vi "HFRR ADV v038.vi"() -> ()   [LabVIEW 2025] (continued)
    n1685 = case shown="True" w2039 {
      selector: w2039 -> [_ w2047]
      tunnel: w2037 -> [_ w2048]
      frame False {
      }
      frame True {
        n1686 = Not(x=w2047) -> (.not. x?=w2046:bool)
        n1687 = local write "Calibration Tare"(w2046) -> ()
        "Calibration Tare Value" <- w2048
      }
    }
    n1688 = local read "Quit"() -> (w2045:bool)
  }
  n1689 = while {
    stop <- w2071 stop-if-true
    n1690 = local read "Due read"() -> (w2069:string)
    n1691 = call <vilib>:"High Resolution Polling Wait.vi"("seconds to wait"=0.02) -> ()  [unwired: 10 in, 1 out]
    n1692 = local read "Frictioin Force Raw"() -> (w2051:dbl)
    n1693 = Spreadsheet String To Array(delimiter (Tab)=";", format string="", spreadsheet string=w2069, array type (2D Dbl)=string[] []) -> (array=w2066:string[])
    n1694 = Fract/Exp String To Number(string=w2066) -> (number=w2065:dbl[])  [unwired: 3 in, 1 out]
    n1695 = call <vilib>:"Median Filter PtByPt.vi"("rank"=2, "x"=w2051) -> ("Filtered x"=→"Friction":dbl)  [unwired: 2 in, 1 out]
    n1696 = Index Array(array=w2065) -> (element #1=→"Sample Temperature":dbl, element #2=→"Target Sample Temperature":dbl, element #3=→"Current Duty Cycle":dbl, element #4=→"Ambient Temperature":dbl, element #5=→"Dac Status":dbl, element #6=→"Vpp":dbl, element #7=→"Active Error Code":dbl, element #8=→"Kp":dbl, element #9=→"Ki":dbl, element #10=→"Kd":dbl, element #11=→"SampleRaw":dbl, element #12=→"AmbRaw":dbl)  [unwired: 12 in]
    n1697 = local read "Quit"() -> (w2071:bool)
  }
  n1698 = while {
    shift-right: [w2085] -> w41
    shift-left: _ -> [w2077]
    shift-right: [w2072] -> w40
    shift-left: errorcluster {"status"=FALSE, "code"=0, "source"="Init"} ("error out") -> [w2079]
    tunnel: [w2074] -> w44
    tunnel: [w2084] -> _
    i -> [w2084]
    stop <- w2074 stop-if-true
    n1699 = local read "Com Port 2"() -> (w2078:refnum<visa-resource-name>)
    n1700 = local read "Port 2a"() -> (w2080:bool)
    n1701 = Unbundle(w2079) -> ("status"=→"Port 4":bool)  [unwired: 2 out]
    n1702 = call <vilib>:"High Resolution Polling Wait.vi"("seconds to wait"=0.02) -> ()  [unwired: 10 in, 1 out]
    n1703 = local read "Port 4"() -> (w2081:bool)
    n1704 = Not Equal?(x=w2078, y=w2077) -> (x != y?=w2076:bool)
    n1705 = Or(x=w2081, y=w2080) -> (x .or. y?=w2083:bool)
    n1706 = case shown="False" w2083 {
      frame False {
        w2088 = TRUE ("Visible")
        n1707 = property on="Port 2a" class="Bool (strict)"("Visible"=w2088) -> ()  [unwired: 2 in, 2 out]
        n1708 = property on="Port 4" class="Bool (strict)"("Visible"=w2088) -> ()  [unwired: 2 in, 2 out]
      }
      frame True {
        w2089 = TRUE ("Visible")
        n1709 = property on="Port 2a" class="Bool (strict)"("Visible"=w2089) -> ()  [unwired: 2 in, 2 out]
        n1710 = property on="Port 4" class="Bool (strict)"("Visible"=w2089) -> ()  [unwired: 2 in, 2 out]
      }
    }
    n1711 = case shown="True" w2076 {
      tunnel: [w2086 errorcluster {"status"=TRUE, "code"=0, "source"="Init"} ("error out")] -> w2075
      tunnel: w2079 -> [w2086 _]
      frame False {
      }
      frame True {
      }
    }
    n1712 = case shown="No Error" w2075 {
      selector: w2075 -> [w2102 w2133]
      tunnel: [w2095 w2138] -> w2085
      tunnel: [w2103 w2131] -> w2072
      tunnel: w2077 -> [w2104 w2136]
      frame No Error {
        n1713 = property class="Instr" props=["Serial Settings:Number of Bytes at Serial Port"](reference=w2104, error in=w2102) -> (reference out=w2096:refnum<visa-resource-name>, error out=w2101:errorcluster)  [unwired: 1 out]
        n1714 = while {
          tunnel: [w2112] -> w2097
          tunnel: [w2111] -> w2098
          tunnel: w2101 -> [w2110]
          tunnel: w2096 -> [w2109]
          tunnel: [w2108] -> _
          i -> [w2108]
          stop <- TRUE stop-if-true
          n1715 = property class="Instr" props=["Serial Settings:Number of Bytes at Serial Port"](reference=w2109, error in=w2110) -> (reference out=w2114:refnum<visa-resource-name>, error out=w2113:errorcluster)  [unwired: 1 out]
          n1716 = VISA Read(VISA resource name=w2114, byte count=u32 1000, error in (no error)=w2113) -> (VISA resource name out=w2111:refnum<visa-resource-name>, read buffer=→"Due read":string, error out=w2112:errorcluster)  [unwired: 1 out]
        }
        n1717 = local read "Due Write"() -> (w2094:string)
        n1718 = call <vilib>:"Trim Whitespace.vi"("string"=w2094) -> ("trimmed string"=w2093:string)  [unwired: 1 in]
        n1719 = Not Equal?(x=w2093, y="") -> (x != y?=w2099:bool)
        n1720 = VISA Flush I/O Buffer(VISA resource name=w2098) -> (VISA resource name out=w2091:refnum<visa-resource-name>, error out=→"error out 10":errorcluster)  [unwired: 2 in]
        n1721 = case shown="True" w2099 {
          tunnel: w2091 -> [w2116 w2121]
          tunnel: [w2116 w2125] -> w2095
          tunnel: w2097 -> [w2115 w2120]
          tunnel: [w2115 w2123] -> w2103
          tunnel: w2093 -> [_ w2119]
          tunnel: [_ w2122] -> _
          frame False {
            # "DATA  WRITE LOOP"
          }
          frame True {
            n1722 = Concatenate Strings(w2119, "\r\n") -> (w2118:string)
            n1723 = VISA Write(VISA resource name=w2121, write buffer=w2118, error in (no error)=w2120) -> (VISA resource name out=w2125:refnum<visa-resource-name>, return count=w2122:u32, error out=w2124:errorcluster)
            n1724 = flat-sequence {
              tunnel: w2124 -> [w2127]
              tunnel: [w2127] -> w2123
              frame #0 {
                n1725 = local write "Due Write"("" ("Command")) -> ()
                n1726 = Wait (ms)(milliseconds to wait=u32 5) -> ()  [unwired: 1 out]
              }
            }
          }
        }
        "Port 2a" <- TRUE ("Port 2a")
      }
      frame Error {
        w2144 = u16 0 items=["None", "XON/XOFF", "RTS/CTS", "XON/XOFF & RTS/CTS", "DTR/DSR", "XON/XOFF & DTR/DSR"] ("flow control (0:none)  2")
        w2142 = u16 10 items=["1.0"=10, "1.5"=15, "2.0"=20] ("stop bits 2")
        w2140 = u16 0 items=["None", "Odd", "Even", "Mark", "Space"] ("parity 2")
        w2141 = u32 10000  # timeout (10sec)
        n1727 = VISA Clear(VISA resource name=w2136, error in (no error)=w2133) -> (VISA resource name out=w2135:refnum<visa-resource-name>, error out=w2134:errorcluster)
        n1728 = VISA Close(VISA resource name=w2135, error in (no error)=w2134) -> (error out=w2137:errorcluster)
        n1729 = call <vilib>:"Clear Errors.vi"("error in (no error)"=w2137) -> ()  [unwired: 5 in, 2 out]
        n1730 = local write "Port 2a"(FALSE ("Port 2a")) -> ()
        n1731 = local read "Com Port 2"() -> (w2130:refnum<visa-resource-name>)
        "visa due" <- w2130
        n1732 = call-poly "VISA Configure Serial Port"("VISA resource name"=w2130, "timeout (10sec)"=w2141, "baud rate (9600)"=u32 250000 ("baud rate  2"), "data bits (8)"=u16 8 ("data bits  2"), "parity (0:none)"=w2140, "stop bits (10: 1 bit)"=w2142, "flow control (0:none)"=w2144) -> ("VISA resource name out"=w2145:refnum<visa-resource-name>, "error out"=w2146:errorcluster)  [unwired: 7 in]
        n1733 = flat-sequence {
          tunnel: w2145 -> [w2148]
          tunnel: w2146 -> [w2147]
          tunnel: [w2148] -> w2138
          tunnel: [w2147] -> w2131
          frame #0 {
            n1734 = Wait (ms)(milliseconds to wait=u32 50) -> ()  [unwired: 1 out]
          }
        }
        "Residual Due" <- ""
      }
    }
    "error out 9" <- w2072
    n1735 = local read "Quit"() -> (w2074:bool)
    "Error Due" <- w2079
  }
  n1736 = local write "FRICVALZ"(0.0 ("FRICVALZ")) -> ()
  n1737 = property on="RUN" class="Bool (strict)"("Visible"=TRUE) -> ()  [unwired: 2 in, 2 out]
  n1738 = while {
    tunnel: [w2163] -> _
    tunnel: [w2150] -> w54
    i -> [w2163]
    stop <- w2150 stop-if-true
    n1739 = local read "conststatus"() -> (w2154:dbl)
    n1740 = local read "Main Tab"() -> (w2152:T2)
    n1741 = local read "EDIT"() -> (w2169:bool)
    n1742 = local read "Rate"() -> (w2168:dbl)
    n1743 = case shown="True" w2169 {
      tunnel: [FALSE TRUE] -> _
      frame False {
      }
      frame True {
      }
    }
    n1744 = Equal?(x=w2152, y=T29."About" ("Main Tab")) -> (x = y?=w2161:bool)
    n1745 = Equal?(x=w2154, y=0.0) -> (x = y?=w2155:bool)
    n1746 = Divide(x=1.0, y=w2168) -> (x/y=w2164:dbl)
    "Time 2" <- w2164
    n1747 = case shown="True" w2155 {
      frame False {
      }
      frame True {
        # "C:\\WinDucom\\calibrate WO 2391.dcf"
        n1748 = local write "Lan flag"(22) -> ()
        n1749 = local write "conststatus"(10.0 ("rpm value : 2")) -> ()
        n1750 = String To Path(string="C:\\LAB-IQ\\calibrate WO 2465.dcf") -> (path=w2175:path)
        n1751 = Open/Create/Replace File "Open File"(file path (use dialog)=w2175) -> (refnum out=w2173:refnum<file>)  [unwired: 5 in, 2 out]
        n1752 = for {
          N: 23 -> [_]
          tunnel: w2173 -> [w2184]
          i -> [w2178]
          (unwired) TRUE ("line mode (F)")
          n1753 = Read from Text File "Read File"(file (use dialog)=w2184) -> (text=w2183:string)  [unwired: 3 in, 3 out]
          n1754 = Match Pattern(string=w2183, regular expression="]") -> (after substring=w2181:string)  [unwired: 1 in, 3 out]
          n1755 = String Subset(string=w2183, offset (0)=5, length (rest)=10 ("length (rest)")) -> (substring=w2176:string)
          n1756 = Fract/Exp String To Number(string=w2176) -> (number=w2177:dbl)  [unwired: 3 in, 1 out]
          n1757 = Match Pattern(string=w2181, regular expression="-") -> (before substring=w2179:string)  [unwired: 1 in, 3 out]
          n1758 = case shown="10" w2178 {
            tunnel: w2177 -> [_ _ _ _ _ _ _ _ _ _ w2191 _ _ _ _ _ _ _ _ _ _ _ _ _]
            tunnel: w2179 -> [_ _ _ _ w2187 w2188 w2189 _ _ _ _ _ _ _ _ _ _ _ _ _ w2192 w2193 w2194 _]
            frame 0 {
            }
            frame 1 {
            }
            frame 2 {
            }
            frame 3 {
            }
            frame 4 {
              n1759 = local write "Com Port 1"(w2187) -> ()
            }
            frame 5 {
              n1760 = local write "Com Port 2"(w2188) -> ()
              n1761 = local write "visa due"(w2188) -> ()
            }
            frame 6 {
              n1762 = String To Path(string=w2189) -> (path=w2190:path)
              n1763 = local write "File Path"(w2190) -> ()
              "String" <- w2189
            }
            frame 7 {
            }
            frame 8 {
            }
            frame 9 {
            }
            frame 10 {
              n1764 = local write "Language Selection"(w2191) -> ()
            }
            frame 11 {
            }
            frame 12 {
            }
            frame 13 {
            }
            frame 14 {
            }
            frame 15 {
            }
            frame 16 {
            }
            frame 17 {
            }
            frame 18 {
            }
            frame 21 {
            }
            frame 22 {
              n1765 = local write "Com Port 3"(w2192) -> ()
            }
            frame 20 {
              n1766 = local write "Camera Port :"(w2193) -> ()
            }
            frame 19 {
              n1767 = local write "C3 :"(w2194) -> ()
            }
            frame 23, Default {
            }
          }
        }
      }
    }
    n1768 = Select(t=u32 2500 ("milliseconds to wait"), s=w2161, f=u32 500 ("milliseconds to wait")) -> (s? t:f=w2159:u32)
    n1769 = Multiply(x=w2164, y=w2159) -> (x*y=w2166:dbl)
    n1770 = call "Elapsed Time2"("Time Target (s)"=w2166, "Auto Reset"=TRUE) -> ("Time has Elapsed"=w2156:bool)  [unwired: 10 in, 7 out]
    n1771 = case shown="True" w2156 {
      frame False {
      }
      frame True {
        n1772 = stacked-sequence {
          frame #0 {
            # "DATA PROCESSING"
            # "115 mV/N"
            n1773 = local read "Sample Temperature"() -> (w2197:dbl)
            n1774 = local read "RH Numeric:"() -> (→"Humidity ( %RH )":dbl)
            n1775 = local read "FRICVALZ"() -> (w2214:dbl)
            n1776 = local read "Friction"() -> (w2200:dbl)
            n1777 = call <vilib>:"Mean PtByPt.vi"("x"=w2197, "sample length"=100) -> ("mean"=w2196:dbl)  [unwired: 2 in, 1 out]
            "TEMP 2" <- w2196
            "TEMP 3" <- w2196
            n1778 = Subtract(x=w2200, y=w2214) -> (x-y=w2209:dbl)
            "FF 2" <- w2209
            "FF 4" <- w2209
            n1779 = local read "Ambient Temperature"() -> (→"AIR TEMP":dbl)
            n1780 = local read "TEMP"() -> (w2213:dbl)
            n1781 = local write "FF 3"(w2209) -> ()
            n1782 = Compound Arithmetic op=OR("FRICVALZ 4", "FRICVALZ 3", "FRICVALZ 2") -> (w2205:bool)
            n1783 = case shown="True" w2205 {
              tunnel: w2200 -> [_ w2220]
              frame False {
              }
              frame True {
                w2219 = FALSE ("FRICVALZ")
                n1784 = local write "FRICVALZ 3"(w2219) -> ()
                n1785 = local write "FRICVALZ 2"(w2219) -> ()
                n1786 = local write "FRICVALZ 4"(w2219) -> ()
                "FRICVALZ" <- w2220
              }
            }
            n1787 = Not A Number/Path/Refnum?(number/path/refnum=w2213) -> (NaN/Path/Refnum?=w2212:bool)
            n1788 = Not A Number/Path/Refnum?(number/path/refnum=w2209) -> (NaN/Path/Refnum?=w2211:bool)
            n1789 = Divide(x=w2209, y=1.96) -> (x/y=w2206:dbl)
            n1790 = Compound Arithmetic op=OR(w2212, w2211) -> (w2210:bool)
            n1791 = Not A Number/Path/Refnum?(number/path/refnum=w2206) -> (NaN/Path/Refnum?=w2207:bool)
            n1792 = case shown="True" w2210 {
              frame False {
              }
              frame True {
                n1793 = local write "TEMP"(0.0 ("TEMP")) -> ()
                n1794 = local write "FF 2"(0.0 ("FF 2")) -> ()
                n1795 = local write "reinit"(TRUE ("reinit")) -> ()
              }
            }
            n1796 = local write "TEMP"(w2196) -> ()
            n1797 = Select(t=0.0, s=w2207, f=w2206) -> (s? t:f=w2199:dbl)
            "COF 2" <- w2199
            n1798 = local write "COF 3"(w2199) -> ()
          }
        }
      }
    }
    n1799 = Wait (ms)(milliseconds to wait=u32 50) -> ()  [unwired: 1 out]
    n1800 = local read "Quit"() -> (w2150:bool)
    "Rate" <- 2500.0 ("No of Samples")
  }
  n1801 = while {
    tunnel: [w2240] -> _
    tunnel: [w2223] -> w56
    tunnel: w1 -> [_]
    i -> [w2240]
    stop <- w2223 stop-if-true
    # "C:\\LAB-IQ-NXT\\Scar View.exe"
    n1802 = local read "OK Button 16"() -> (w2230:bool)
    n1803 = local read "Main Tab"() -> (w2224:T2)
    n1804 = local read "service 3"() -> (w2225:bool)
    n1805 = local read "OPEN 6"() -> (w2227:bool)
    n1806 = local read "EDIT 2"() -> (w2229:bool)
    n1807 = flat-sequence {
      frame #0 {
        n1808 = stacked-sequence {
          frame #0 {
            n1809 = local read "EDIT"() -> (w2718:bool)
            n1810 = case shown="False" w2718 {
              tunnel: [u8 2 ("Disabled") u8 0 ("Disabled")] -> _
              frame False {
                w2720 = FALSE
                n1811 = local write "Password"("") -> ()
                n1812 = local write "x = y?"(w2720) -> ()
                n1813 = property on="Password" class="Str"("Visible"=w2720) -> ()  [unwired: 2 in, 2 out]
              }
              frame True {
                n1814 = property on="Password" class="Str"("Visible"=TRUE) -> ()  [unwired: 2 in, 2 out]
              }
            }
            "dipl pwd" <- "@143$\n" ("dipl pwd")
          }
          frame #1 {
          }
          frame #2 {
          }
          frame #3 {
          }
          frame #4 {
            n1815 = String To Byte Array(string="Password") -> (unsigned byte array=w2731:u8[])
            n1816 = Search 1D Array(1D array=w2731, element=u8 10) -> (index of element=w2729:i32)  [unwired: 1 in]
            n1817 = Index Array(array=w2731, index=w2729) -> (element=w2730:u8)
            n1818 = Equal?(x=w2730, y=10) -> (x = y?=w2726:bool)
            n1819 = case shown="True" w2726 {
              frame False {
              }
              frame True {
                # "password"
                # "password"
                n1820 = local read "Password"() -> (w2743:string)
                n1821 = String To Byte Array(string=w2743) -> (unsigned byte array=w2746:u8[])
                n1822 = String To Byte Array(string="@143$\n") -> (unsigned byte array=w2733:u8[])
                n1823 = Array Size(array=w2746) -> (size(s)=w2742:i32)
                n1824 = Array Size(array=w2733) -> (size(s)=w2738:i32)
                n1825 = for {
                  N: w2742 -> [_]
                  tunnel: w2746 -> [w2759]
                  tunnel: [w2757] -> w2747 mode=indexing
                  tunnel: w2742 -> [w2754]
                  i -> [w2755]
                  n1826 = Decrement(x=w2754) -> (x-1=w2753:i32)
                  n1827 = Index Array(array=w2759, index=w2755) -> (element=w2758:u8)
                  n1828 = Equal?(x=w2755, y=w2753) -> (x = y?=w2752:bool)
                  n1829 = Number To Decimal String(number=w2758) -> (decimal integer string=w2756:string)  [unwired: 1 in]
                  n1830 = Select(t="", s=w2752, f="\r") -> (s? t:f=w2749:string)
                  n1831 = Concatenate Strings(w2756, w2749) -> (w2757:string)
                }
                n1832 = for {
                  N: w2738 -> [_]
                  tunnel: w2733 -> [w2770]
                  tunnel: [w2768] -> w2736 mode=indexing
                  tunnel: w2738 -> [w2765]
                  i -> [w2766]
                  n1833 = Decrement(x=w2765) -> (x-1=w2764:i32)
                  n1834 = Index Array(array=w2770, index=w2766) -> (element=w2769:u8)
                  n1835 = Equal?(x=w2766, y=w2764) -> (x = y?=w2763:bool)
                  n1836 = Number To Decimal String(number=w2769) -> (decimal integer string=w2767:string)  [unwired: 1 in]
                  n1837 = Select(t="", s=w2763, f="\r") -> (s? t:f=w2760:string)
                  n1838 = Concatenate Strings(w2767, w2760) -> (w2768:string)
                }
                n1839 = local read "file path"() -> (w2732:path)
                n1840 = call <vilib>:"Read Characters From File.vi"("file path (dialog if empty)"=w2732) -> ("character string"=w2745:string)  [unwired: 5 in, 3 out]
                "string" <- w2745
                n1841 = flat-sequence {
                  tunnel: [w2748] -> _
                  frame #0 {
                    w2748 = ""
                    n1842 = local write "Password"(w2748) -> ()
                  }
                }
                n1843 = Concatenate Strings(w2736) -> (w2737:string)
                n1844 = Concatenate Strings(w2745) -> (w2744:string)
                n1845 = Concatenate Strings(w2747) -> (w2740:string)
                n1846 = Equal?(x=w2740, y=w2744) -> (x = y?=w2735:bool)
                n1847 = Equal?(x=w2740, y=w2737) -> (x = y?=w2741:bool)
                n1848 = Or(x=w2735, y=w2741) -> (x .or. y?=→"x = y?":bool)
              }
            }
          }
        }
        n1849 = local read "x = y?"() -> (w2716:bool)
        n1850 = And(x="EDIT", y=w2716) -> (x .and. y?=w2714:bool)
        n1851 = case shown="True" w2714 {
          tunnel: [u8 2 ("Disabled") u8 0 ("Disabled")] -> w2713
          tunnel: [w2920 TRUE ("Visible")] -> w2712
          frame False {
            w2920 = FALSE ("Visible")
            n1852 = local write "EDIT 2"(w2920) -> ()
          }
          frame True {
          }
        }
        n1853 = case shown="True" "SAVE" {
          frame False {
          }
          frame True {
            n1854 = stacked-sequence {
              seq-local: [w2775 _ _] -> [_ w2916 _]
              frame #0 {
                w2771 = 0.0 ("number")
                w2772 = 0.0 ("number")
                (unwired) i16 5 ("precision (6)")
                # "[CH1]    - FF\n[CH2]   - TEMPERATURE\n[CH3]    - Humidity\n[CH4]    - AIR TEMP\n[CH5]\\- Visa Uno\n[CH6] \\- Visa Due\n[CH7]  \\- file path\n[CH8]   - Displacement Gain\n[CHA]   - Stroke Gain\n[CHB]   - Stroke PID Gain\n[CHC]   -Language Selection\n[CHD]   -Power +\n[CHE]   -Power_\n[CHF]   -Heater\n[CHG]   -Humidity Wet\n[CHH]   -Humidity Dry\n[CHI]   -Integral Time"
                n1855 = local read "Language Selection"() -> (w2818:enum16{"English", "Russian"})
                n1856 = Path To String(path="File Path") -> (string=w2834:string)
                n1857 = Number To Fractional String(number=w2771, width (-)=i16 10 ("precision (6)"), precision (6)=i16 5) -> (F-format string=w2825:string)  [unwired: 1 in]
                n1858 = Number To Fractional String(number=w2818, width (-)=i16 10 ("precision (6)"), precision (6)=i16 5) -> (F-format string=w2814:string)  [unwired: 1 in]
                n1859 = Number To Fractional String(number=w2772, width (-)=i16 10 ("precision (6)"), precision (6)=i16 5) -> (F-format string=w2808:string)  [unwired: 1 in]
                n1860 = Number To Fractional String(number=w2772, width (-)=i16 10 ("precision (6)"), precision (6)=i16 5) -> (F-format string=w2805:string)  [unwired: 1 in]
                n1861 = Number To Fractional String(number=w2772, width (-)=i16 10 ("precision (6)"), precision (6)=i16 5) -> (F-format string=w2800:string)  [unwired: 1 in]
                n1862 = Number To Fractional String(number=w2772, width (-)=i16 10 ("precision (6)"), precision (6)=i16 5) -> (F-format string=w2797:string)  [unwired: 1 in]
                n1863 = Number To Fractional String(number=w2772, width (-)=i16 10 ("precision (6)"), precision (6)=i16 5) -> (F-format string=w2792:string)  [unwired: 1 in]
                n1864 = local read "Com Port 1"() -> (w2774:refnum<visa-resource-name>)
                n1865 = local read "Com Port 2"() -> (w2773:refnum<visa-resource-name>)
                n1866 = Concatenate Strings(w2834, "\\" ("string")) -> (w2833:string)
                n1867 = Number To Fractional String(number=w2771, width (-)=i16 10 ("precision (6)"), precision (6)=i16 5) -> (F-format string=w2866:string)  [unwired: 1 in]
                n1868 = Number To Fractional String(number=w2771, width (-)=i16 10 ("precision (6)"), precision (6)=i16 5) -> (F-format string=w2865:string)  [unwired: 1 in]
                n1869 = Number To Fractional String(number=w2771, width (-)=i16 10 ("precision (6)"), precision (6)=i16 5) -> (F-format string=w2859:string)  [unwired: 1 in]
                n1870 = Number To Fractional String(number=w2771, width (-)=i16 10 ("precision (6)"), precision (6)=i16 5) -> (F-format string=w2853:string)  [unwired: 1 in]
                n1871 = Number To Fractional String(number=w2771, width (-)=i16 10 ("precision (6)"), precision (6)=i16 5) -> (F-format string=w2826:string)  [unwired: 1 in]
                n1872 = Concatenate Strings("[CHA]" ("string"), w2825, "- Stroke Gain" ("string"), "\r") -> (w2819:string)
                n1873 = Concatenate Strings("[CHC]" ("string"), w2814, "-Language Selection" ("string"), "\r") -> (w2811:string)
                n1874 = Concatenate Strings("[CHD]" ("string"), w2808, "-Power +" ("string"), "\r") -> (w2790:string)
                n1875 = Concatenate Strings("[CHG]" ("string"), w2797, "-Humidity Wet" ("string"), "\r") -> (w2787:string)
                n1876 = Concatenate Strings("[CHH]" ("string"), w2792, "-Humidity Dry" ("string"), "\r") -> (w2786:string)
                n1877 = Concatenate Strings("[CH1]" ("string"), w2866, " - FF" ("string"), "\r") -> (w2864:string)
                n1878 = Concatenate Strings("[CH2]" ("string"), w2865, " - TEMPERATURE" ("string"), "\r") -> (w2863:string)
                n1879 = Concatenate Strings("[CH3]" ("string"), w2859, " - Humidity" ("string"), "\r") -> (w2856:string)
                n1880 = Concatenate Strings("[CH4]" ("string"), w2853, " - AIR TEMP" ("string"), "\r") -> (w2849:string)
                n1881 = Concatenate Strings("[CH5]" ("string"), w2774, "- Visa Uno" ("string"), "\r") -> (w2842:string)
                n1882 = Concatenate Strings("[CH6]" ("string"), w2773, "- Visa Due" ("string"), "\r") -> (w2837:string)
                n1883 = Concatenate Strings("[CH7]" ("string"), w2833, "- file path" ("string"), "\r") -> (w2836:string)
                n1884 = Concatenate Strings("[CH8]" ("string"), w2826, "- Displacement Gain" ("string"), "\r") -> (w2829:string)
                n1885 = Concatenate Strings("[CHE]" ("string"), w2805, "-Power_" ("string"), "\r") -> (w2789:string)
                n1886 = Concatenate Strings("[CHF]" ("string"), w2800, "-Heater" ("string"), "\r") -> (w2788:string)
                n1887 = Concatenate Strings(w2864, w2863, w2856, w2849, w2842, w2837, w2836, w2829, w2819, w2811, w2790, w2789, w2788, w2787, w2786) -> (w2775:string)
                "gain" <- w2775
              }
              frame #1 {
                w2877 = 0.0 ("number")
                n1888 = local read "Camera Port :"() -> (w2880:string)
                n1889 = local read "C3 :"() -> (w2888:refnum<visa-resource-name>)
                n1890 = local read "Com Port 3"() -> (w2889:refnum<visa-resource-name>)
                n1891 = Concatenate Strings("[CH8]" ("string"), w2880, "- Visa Camera" ("string"), "\r") -> (w2879:string)
                n1892 = Concatenate Strings("[CH7]" ("string"), w2888, "- Visa Humidity" ("string"), "\r") -> (w2884:string)
                n1893 = Number To Fractional String(number=w2877, width (-)=i16 10 ("precision (6)"), precision (6)=i16 5) -> (F-format string=w2904:string)  [unwired: 1 in]
                n1894 = Concatenate Strings("[CHL]" ("string"), w2889, "- Visa humid" ("string"), "\r") -> (w2892:string)
                n1895 = Number To Fractional String(number=w2877, width (-)=i16 10 ("precision (6)"), precision (6)=i16 5) -> (F-format string=w2911:string)  [unwired: 1 in]
                n1896 = Concatenate Strings("[CHK]" ("string"), w2904, "-TEMP INTERCEPT" ("string"), "\r") -> (w2900:string)
                n1897 = Concatenate Strings("[SNO]" ("string"), "" ("string"), "-" ("string"), "\r") -> (w2897:string)
                n1898 = Concatenate Strings("[CHJ]" ("string"), w2911, "-AIR TEMP INTERCEPT" ("string"), "\r") -> (w2901:string)
                n1899 = String To Path(string="C:\\LAB-IQ\\calibrate WO 2465.dcf") -> (path=w2890:path)
                n1900 = Concatenate Strings(w2916, w2901, w2900, w2897, w2892, w2884, w2879) -> (w2915:string)
                n1901 = call <vilib>:"Write Characters To File.vi"("append to file? (new file:F)"=FALSE, "character string"=w2915, "file path (dialog if empty)"=w2890) -> ()  [unwired: 2 in, 1 out]
              }
              frame #2 {
                n1902 = local write "Lan flag"(0.0 ("Lan flag")) -> ()
                n1903 = local write "conststatus"(0.0 ("rpm value : 2")) -> ()
                n1904 = local write "SAVE"(FALSE ("OK Button 14")) -> ()
              }
            }
          }
        }
        n1905 = property on="EDIT 2" class="Bool (strict)"("Visible"=w2712) -> ()  [unwired: 2 in, 2 out]
        n1906 = property on="SAVE" class="Bool (strict)"("Visible"=w2712) -> ()  [unwired: 2 in, 2 out]
        n1907 = property on="visa due" class="CmbBox"("Disabled"=w2713) -> ()  [unwired: 2 in, 2 out]
        n1908 = property on="File Path" class="Path"("Disabled"=w2713) -> ()  [unwired: 2 in, 2 out]
        n1909 = property on="Language Selection" class="Enum (strict)"("Visible"=w2712) -> ()  [unwired: 2 in, 2 out]
        n1910 = property on="SPEED OUT:" class="DigNum (strict)"("Disabled"=w2713) -> ()  [unwired: 2 in, 2 out]
      }
    }
    n1911 = local read "RUN"() -> (w2239:bool)
    n1912 = local read "RUN"() -> (w2237:bool)
    n1913 = case shown="True" "EDIT 3" {
      frame False {
      }
      frame True {
        n1914 = local write "EDIT 3"(FALSE ("EDIT 3")) -> ()
        n1915 = local write "Main Tab"(T2."About" ("Main Tab")) -> ()
      }
    }
    n1916 = case shown="False" w2239 {
      frame False {
        n1917 = local read "stopT"() -> (w2927:bool)
        n1918 = case shown="True" w2927 {
          frame False {
          }
          frame True {
            n1919 = local write "stopT"(FALSE) -> ()
          }
        }
      }
      frame True {
        "stopT" <- TRUE
      }
    }
    n1920 = case shown="False" w2237 {
      frame False {
      }
      frame True {
      }
    }
    n1921 = case shown="True" w2229 {
      frame False {
        n1922 = property on="Password 2" class="Str"("Visible"=FALSE) -> ()  [unwired: 2 in, 2 out]
        n1923 = local write "Password 2"("" ("Password")) -> ()
      }
      frame True {
        n1924 = property on="Password 2" class="Str"("Visible"=TRUE) -> ()  [unwired: 2 in, 2 out]
        n1925 = Equal?(x="Password 2", y="HFRR1234") -> (x = y?=w2252:bool)
        n1926 = case shown="True" w2252 {
          tunnel: "Password 2" -> [w2255 _]
          frame False {
            n1927 = String Length(string=w2255) -> (length=w2256:i32)
            n1928 = Greater Than 0?(x=w2256) -> (x > 0?=w2254:bool)
            n1929 = case shown="False" w2254 {
              frame False {
                n1930 = property on="Password 2" class="Str"("Caption.Text"="Password (Advance Setting)") -> ()  [unwired: 2 in, 2 out]
              }
              frame True {
                n1931 = property on="Password 2" class="Str"("Caption.Text"="Incorrect Password!") -> ()  [unwired: 2 in, 2 out]
              }
            }
          }
          frame True {
            n1932 = local write "EDIT 2"(FALSE ("EDIT 2")) -> ()
            n1933 = local write "Password 2"("" ("Password")) -> ()
            n1934 = local write "Main Tab"(T2."Advance" ("Main Tab")) -> ()
            n1935 = local write "Main Dashboard Buttons"(T1."Advance" ("Main Dashboard Buttons")) -> ()
          }
        }
      }
    }
    n1936 = case shown="True" "Prog Uno" {
      frame False {
      }
      frame True {
        n1937 = stacked-sequence {
          frame #0 {
            n1938 = Delete(path (use dialog)=path "C:/LAB-IQ-NXT/UNOCOMPILE.bat" ("working directory")) -> ()  [unwired: 4 in, 3 out]
          }
          frame #1 {
            n1939 = local read "Com Port 1"() -> (w2694:refnum<visa-resource-name>)
            n1940 = Concatenate Strings("cmd.exe /c \"mode " ("command line"), w2694, ":1200,n,8,1\"\n" ("command line")) -> (w2699:string)
            n1941 = Concatenate Strings(w2699, "CD\\\nCD WinDucom\navrdude -C avrdude.conf -v -patmega328p -carduino -P" ("command line"), w2694, " -b115200 -D -Uflash:w:UNO_V20.hex:i\n" ("command line"), "\r") -> (w2701:string)
            "STR" <- w2701
            n1942 = call <vilib>:"Write Characters To File.vi"("append to file? (new file:F)"=FALSE, "character string"=w2701, "file path (dialog if empty)"=path "C:/LAB-IQ/UNOCOMPILE.bat" ("working directory")) -> ()  [unwired: 2 in, 1 out]
          }
          frame #2 {
            n1943 = disable-structure shown="Disabled" {
              frame Disabled {
                w2705 = "cmd.exe  /c \"C:\\LAB-IQ-NXT\\UNOCOMPILE.bat\"" ("string")
                n1944 = local write "Prog Uno"(FALSE ("run minimized? (F)")) -> ()
                n1945 = call <vilib>:"System Exec.vi"("expected output size  (4096)"=u32 65535, "run minimized? (F)"=FALSE, "wait until completion? (T)"=TRUE ("run minimized? (F)"), "working directory"=path "C:/LAB-IQ-NXT", "standard input"=w2705, "command line"=w2705) -> ("error out"=w2704:errorcluster, "standard output"=→"String 42":string)  [unwired: 2 in, 2 out]
                "error out 3" <- w2704
                n1946 = flat-sequence {
                  tunnel: w2704 -> [_]
                  frame #0 {
                  }
                }
              }
              frame Enabled {
              }
            }
          }
        }
      }
    }
    n1947 = case shown="\"ISO 12156\"" "TEST STANDARD" {
      frame "ASTM D6079", Default {
        w2674 = 50.0 ("Hz")
        w2675 = 53.0 ("Set Rh")
        w2677 = 1.0 ("Set Strk")
        w2676 = 60.0 ("Set Temp")
        # "astm hide"
        n1948 = local write "NORMAL LOAD"(200.0 ("NORMAL LOAD")) -> ()
        n1949 = local write "Set Strk"(w2677) -> ()
        n1950 = local write "Set Hz"(w2674) -> ()
        n1951 = local write "Set Temp"(w2676) -> ()
        n1952 = local write "Set Rh"(w2675) -> ()
        n1953 = local write "test time"(75.0 ("test time")) -> ()
        n1954 = local write "Set Stroke:"(w2677) -> ()
        n1955 = local write "Set Humidity:"(w2675) -> ()
        n1956 = local write "Set Frequency:"(w2674) -> ()
        n1957 = local write "Set Temperature:"(w2676) -> ()
        "Test Standard" <- "ASTM D6079" ("Test Standard 2")
      }
      frame "ISO 12156" {
        n1958 = local write "Set Strk"(1.0 ("Set Strk")) -> ()
        n1959 = local write "NORMAL LOAD"(200.0 ("NORMAL LOAD")) -> ()
        n1960 = local write "Set Temp"(60.0 ("Set Temp")) -> ()
        n1961 = local write "test time"(75.0 ("test time")) -> ()
        n1962 = local write "Set Hz"(50.0 ("Hz")) -> ()
        n1963 = local write "Set Rh"(53.0 ("Set Rh")) -> ()
      }
      frame "CEC F-096-A-06" {
        n1964 = local write "Set Strk"(1.0 ("Set Strk")) -> ()
        n1965 = local write "NORMAL LOAD"(200.0 ("NORMAL LOAD")) -> ()
        n1966 = local write "Set Temp"(60.0 ("Set Temp")) -> ()
        n1967 = local write "test time"(75.0 ("test time")) -> ()
        n1968 = local write "Set Hz"(50.0 ("Hz")) -> ()
        n1969 = local write "Set Rh"(53.0 ("Set Rh")) -> ()
      }
      frame "Custom" {
      }
    }
    n1970 = Or(x=w2227, y=w2225) -> (x .or. y?=w2226:bool)
    n1971 = case shown="\"About\"" w2224 {
      tunnel: [T29."Acquire" ("Main Tab") T29."Compare Files" ("Main Tab") T29."About" ("Main Tab")] -> w2235
      frame "Acquire", Default {
      }
      frame "Compare Files" {
      }
      frame "About" {
      }
    }
    n1972 = Or(x=w2230, y="OPEN") -> (x .or. y?=w2231:bool)
    n1973 = case shown="True" w2231 {
      tunnel: w2230 -> [_ w2263]
      frame False {
      }
      frame True {
        n1974 = stacked-sequence {
          tunnel: w2263 -> [_ w2330 _ _]
          frame #0 {
            w2279 = "  " ("String 6")
            n1975 = local write "OPEN"(FALSE ("open")) -> ()
            n1976 = local read "string1 2"() -> (w2267:string)
            n1977 = local read "string1 3"() -> (w2266:string)
            n1978 = local read "string1 4"() -> (w2265:string)
            n1979 = property on="OPEN" class="Bool (strict)"("Visible"=FALSE) -> ()  [unwired: 2 in, 2 out]
            n1980 = local write "String 6"(w2279) -> ()
            n1981 = local write "String 7"(w2279) -> ()
            n1982 = local write "String 8"(w2279) -> ()
            n1983 = local write "String 12"(w2279) -> ()
            n1984 = local read "OK Button 16"() -> (w2264:bool)
            n1985 = String To Path(string=w2267) -> (path=w2275:path)
            n1986 = String To Path(string=w2266) -> (path=w2274:path)
            n1987 = String To Path(string=w2265) -> (path=w2273:path)
            n1988 = case shown="True" w2264 {
              tunnel: [w2280 w2281] -> w2268
              frame False {
                n1989 = local read "string1"() -> (w2280:string)
              }
              frame True {
                n1990 = local read "String Indicator 4"() -> (w2281:string)
              }
            }
            n1991 = Open/Create/Replace File "Open File"(file path (use dialog)=w2275) -> (refnum out=w2271:refnum<file>)  [unwired: 5 in, 2 out]
            n1992 = Open/Create/Replace File "Open File"(file path (use dialog)=w2274) -> (refnum out=w2270:refnum<file>)  [unwired: 5 in, 2 out]
            n1993 = Open/Create/Replace File "Open File"(file path (use dialog)=w2273) -> (refnum out=w2269:refnum<file>)  [unwired: 5 in, 2 out]
            n1994 = while {
              tunnel: w2271 -> [w2293]
              i -> [w2289]
              stop <- w2288 continue-if-true
              (unwired) TRUE ("line mode (F)")
              n1995 = Read from Text File "Read File"(file (use dialog)=w2293) -> (text=w2290:string)  [unwired: 3 in, 3 out]
              n1996 = local write "Numeric 11"(w2289) -> ()
              n1997 = String Length(string=w2290) -> (length=w2292:i32)
              n1998 = Greater?(x=w2292, y=1) -> (0:w2288:bool)
            }
            n1999 = while {
              tunnel: w2270 -> [w2299]
              i -> [w2295]
              stop <- w2294 continue-if-true
              (unwired) TRUE ("line mode (F)")
              n2000 = Read from Text File "Read File"(file (use dialog)=w2299) -> (text=w2296:string)  [unwired: 3 in, 3 out]
              n2001 = local write "Numeric 12"(w2295) -> ()
              n2002 = String Length(string=w2296) -> (length=w2298:i32)
              n2003 = Greater?(x=w2298, y=1) -> (0:w2294:bool)
            }
            n2004 = while {
              tunnel: w2269 -> [w2305]
              i -> [w2301]
              stop <- w2300 continue-if-true
              (unwired) TRUE ("line mode (F)")
              n2005 = Read from Text File "Read File"(file (use dialog)=w2305) -> (text=w2302:string)  [unwired: 3 in, 3 out]
              n2006 = local write "Numeric 13"(w2301) -> ()
              n2007 = String Length(string=w2302) -> (length=w2304:i32)
              n2008 = Greater?(x=w2304, y=1) -> (0:w2300:bool)
            }
            n2009 = String To Path(string=w2268) -> (path=w2276:path)
            n2010 = Open/Create/Replace File "Open File"(file path (use dialog)=w2276) -> (refnum out=w2272:refnum<file>)  [unwired: 5 in, 2 out]
            n2011 = while {
              tunnel: w2272 -> [w2287]
              i -> [w2283]
              stop <- w2282 continue-if-true
              (unwired) TRUE ("line mode (F)")
              n2012 = Read from Text File "Read File"(file (use dialog)=w2287) -> (text=w2284:string)  [unwired: 3 in, 3 out]
              n2013 = local write "Numeric 8"(w2283) -> ()
              n2014 = String Length(string=w2284) -> (length=w2286:i32)
              n2015 = Greater?(x=w2286, y=1) -> (0:w2282:bool)
            }
          }
          frame #1 {
            w2457 = FALSE ("ACTUAL   MERGE")
            # "Sample Temp"
            # "ECR"
            # "COF"
            # "Time\nCOF\nFF\nTemp"
            n2016 = case shown="True" w2330 {
              tunnel: [w2477 w2478] -> w2331
              frame False {
                n2017 = local read "string1"() -> (w2477:string)
              }
              frame True {
                n2018 = local read "String Indicator 4"() -> (w2478:string)
              }
            }
            n2019 = local read "string1 3"() -> (w2375:string)
            n2020 = String To Path(string=w2331) -> (path=w2462:path)
            n2021 = String To Path(string=w2375) -> (path=w2473:path)
            n2022 = local read "Numeric 12"() -> (w2459:i32)
            n2023 = local read "Numeric 8"() -> (w2461:i32)
            n2024 = local read "string1 2"() -> (w2376:string)
            n2025 = local read "string1 4"() -> (w2374:string)
            n2026 = Open/Create/Replace File "Open File"(file path (use dialog)=w2462) -> (refnum out=w2476:refnum<file>, error out=w2475:errorcluster)  [unwired: 5 in, 1 out]
            n2027 = Open/Create/Replace File "Open File"(file path (use dialog)=w2473) -> (refnum out=w2469:refnum<file>, error out=w2470:errorcluster)  [unwired: 5 in, 1 out]
            n2028 = for {
              N: w2461 -> [_]
              tunnel: w2476 -> [w2624]
              tunnel: w2475 -> [w2623]
              tunnel: [w2613] -> w2388 mode=indexing
              tunnel: [w2611] -> w2445 mode=indexing
              tunnel: [w2612] -> w2440 mode=indexing
              tunnel: w2457 -> [_]
              tunnel: [w2605] -> w2442 mode=indexing
              tunnel: [w2601] -> w2411 mode=indexing
              tunnel: [w2597] -> w2386 mode=indexing
              tunnel: [w2593] -> w2367 mode=indexing
              tunnel: [w2588] -> w2327 mode=indexing
              (unwired) TRUE ("line mode (F)")
              # "freq"
              # "Stroke"
              # "Time"
              # "CoF"
              # "Humidity"
              # "Temp"
              # "Air Temp"
              # "ECR"
              n2029 = Read from Text File "Read File"(file (use dialog)=w2624, error in=w2623) -> (text=w2589:string)  [unwired: 2 in, 3 out]
              n2030 = local write "String 6"(w2589) -> ()
              n2031 = String Subset(string=w2589, offset (0)=0, length (rest)=14 ("length (rest)")) -> (substring=w2617:string)
              n2032 = String Subset(string=w2589, offset (0)=35, length (rest)=9 ("length (rest)")) -> (substring=w2614:string)
              n2033 = String Subset(string=w2589, offset (0)=15, length (rest)=9 ("length (rest)")) -> (substring=w2620:string)
              n2034 = Fract/Exp String To Number(string=w2617) -> (number=w2613:dbl)  [unwired: 3 in, 1 out]
              n2035 = Fract/Exp String To Number(string=w2614) -> (number=w2612:dbl)  [unwired: 3 in, 1 out]
              n2036 = Fract/Exp String To Number(string=w2620) -> (number=w2611:dbl)  [unwired: 3 in, 1 out]
              n2037 = String Subset(string=w2589, offset (0)=85, length (rest)=9 ("length (rest)")) -> (substring=w2590:string)
              n2038 = String Subset(string=w2589, offset (0)=25, length (rest)=9 ("length (rest)")) -> (substring=w2596:string)
              n2039 = String Subset(string=w2589, offset (0)=55, length (rest)=9 ("length (rest)")) -> (substring=w2598:string)
              n2040 = String Subset(string=w2589, offset (0)=45, length (rest)=9 ("length (rest)")) -> (substring=w2604:string)
              n2041 = String Subset(string=w2589, offset (0)=65, length (rest)=9 ("length (rest)")) -> (substring=w2610:string)
              n2042 = Fract/Exp String To Number(string=w2596) -> (number=w2593:dbl)  [unwired: 3 in, 1 out]
              n2043 = Fract/Exp String To Number(string=w2590) -> (number=w2588:dbl)  [unwired: 3 in, 1 out]
              n2044 = Fract/Exp String To Number(string=w2598) -> (number=w2597:dbl)  [unwired: 3 in, 1 out]
              n2045 = Fract/Exp String To Number(string=w2604) -> (number=w2601:dbl)  [unwired: 3 in, 1 out]
              n2046 = Fract/Exp String To Number(string=w2610) -> (number=w2607:dbl)  [unwired: 3 in, 1 out]
              n2047 = Add(x=w2607, y=0.0) -> (x+y=w2605:dbl)
            }
            n2048 = for {
              N: w2459 -> [_]
              tunnel: w2470 -> [w2550]
              tunnel: w2469 -> [w2549]
              tunnel: [w2539] -> w2428 mode=indexing
              tunnel: [w2537] -> w2426 mode=indexing
              tunnel: [w2538] -> w2422 mode=indexing
              tunnel: w2457 -> [_]
              tunnel: [w2531] -> w2424 mode=indexing
              tunnel: [w2527] -> w2406 mode=indexing
              tunnel: [w2523] -> w2382 mode=indexing
              tunnel: [w2520] -> w2363 mode=indexing
              tunnel: [w2516] -> w2322 mode=indexing
              (unwired) 9 ("length (rest)")
              (unwired) 9 ("length (rest)")
              (unwired) TRUE ("line mode (F)")
              n2049 = Read from Text File "Read File"(file (use dialog)=w2549, error in=w2550) -> (text=w2517:string)  [unwired: 2 in, 3 out]
              n2050 = local write "String 8"(w2517) -> ()
              n2051 = String Subset(string=w2517, offset (0)=85) -> (substring=w2519:string)  [unwired: 1 in]
              n2052 = String Subset(string=w2517, offset (0)=35, length (rest)=9 ("length (rest)")) -> (substring=w2540:string)
              n2053 = String Subset(string=w2517, offset (0)=55, length (rest)=9 ("length (rest)")) -> (substring=w2525:string)
              n2054 = String Subset(string=w2517, offset (0)=25) -> (substring=w2521:string)  [unwired: 1 in]
              n2055 = String Subset(string=w2517, offset (0)=15, length (rest)=9 ("length (rest)")) -> (substring=w2546:string)
              n2056 = String Subset(string=w2517, offset (0)=0, length (rest)=14 ("length (rest)")) -> (substring=w2543:string)
              n2057 = String Subset(string=w2517, offset (0)=45, length (rest)=9 ("length (rest)")) -> (substring=w2530:string)
              n2058 = String Subset(string=w2517, offset (0)=65, length (rest)=9 ("length (rest)")) -> (substring=w2536:string)
              n2059 = Fract/Exp String To Number(string=w2519) -> (number=w2516:dbl)  [unwired: 3 in, 1 out]
              n2060 = Fract/Exp String To Number(string=w2540) -> (number=w2538:dbl)  [unwired: 3 in, 1 out]
              n2061 = Fract/Exp String To Number(string=w2525) -> (number=w2523:dbl)  [unwired: 3 in, 1 out]
              n2062 = Fract/Exp String To Number(string=w2521) -> (number=w2520:dbl)  [unwired: 3 in, 1 out]
              n2063 = Fract/Exp String To Number(string=w2546) -> (number=w2537:dbl)  [unwired: 3 in, 1 out]
              n2064 = Fract/Exp String To Number(string=w2543) -> (number=w2539:dbl)  [unwired: 3 in, 1 out]
              n2065 = Fract/Exp String To Number(string=w2530) -> (number=w2527:dbl)  [unwired: 3 in, 1 out]
              n2066 = Fract/Exp String To Number(string=w2536) -> (number=w2533:dbl)  [unwired: 3 in, 1 out]
              n2067 = Add(x=w2533, y=0.0) -> (x+y=w2531:dbl)
            }
            n2068 = String To Path(string=w2376) -> (path=w2474:path)
            n2069 = String To Path(string=w2374) -> (path=w2468:path)
            n2070 = local read "Numeric 11"() -> (w2458:i32)
            n2071 = local read "Numeric 13"() -> (w2460:i32)
            n2072 = Open/Create/Replace File "Open File"(file path (use dialog)=w2474) -> (refnum out=w2472:refnum<file>, error out=w2471:errorcluster)  [unwired: 5 in, 1 out]
            n2073 = Open/Create/Replace File "Open File"(file path (use dialog)=w2468) -> (refnum out=w2467:refnum<file>, error out=w2466:errorcluster)  [unwired: 5 in, 1 out]
            n2074 = for {
              N: w2458 -> [_]
              tunnel: w2472 -> [w2587]
              tunnel: w2471 -> [w2586]
              tunnel: [w2576] -> w2438 mode=indexing
              tunnel: [w2574] -> w2436 mode=indexing
              tunnel: [w2575] -> w2431 mode=indexing
              tunnel: w2457 -> [_]
              tunnel: [w2568] -> w2433 mode=indexing
              tunnel: [w2564] -> w2409 mode=indexing
              tunnel: [w2560] -> w2384 mode=indexing
              tunnel: [w2556] -> w2365 mode=indexing
              tunnel: [w2551] -> w2323 mode=indexing
              (unwired) TRUE ("line mode (F)")
              n2075 = Read from Text File "Read File"(file (use dialog)=w2587, error in=w2586) -> (text=w2552:string)  [unwired: 2 in, 3 out]
              n2076 = local write "String 7"(w2552) -> ()
              n2077 = String Subset(string=w2552, offset (0)=85, length (rest)=9 ("length (rest)")) -> (substring=w2555:string)
              n2078 = String Subset(string=w2552, offset (0)=35, length (rest)=9 ("length (rest)")) -> (substring=w2577:string)
              n2079 = String Subset(string=w2552, offset (0)=55, length (rest)=9 ("length (rest)")) -> (substring=w2563:string)
              n2080 = String Subset(string=w2552, offset (0)=25, length (rest)=9 ("length (rest)")) -> (substring=w2557:string)
              n2081 = String Subset(string=w2552, offset (0)=45, length (rest)=9 ("length (rest)")) -> (substring=w2565:string)
              n2082 = String Subset(string=w2552, offset (0)=0, length (rest)=14 ("length (rest)")) -> (substring=w2580:string)
              n2083 = String Subset(string=w2552, offset (0)=15, length (rest)=9 ("length (rest)")) -> (substring=w2583:string)
              n2084 = String Subset(string=w2552, offset (0)=65, length (rest)=9 ("length (rest)")) -> (substring=w2569:string)
              n2085 = Fract/Exp String To Number(string=w2555) -> (number=w2551:dbl)  [unwired: 3 in, 1 out]
              n2086 = Fract/Exp String To Number(string=w2577) -> (number=w2575:dbl)  [unwired: 3 in, 1 out]
              n2087 = Fract/Exp String To Number(string=w2563) -> (number=w2560:dbl)  [unwired: 3 in, 1 out]
              n2088 = Fract/Exp String To Number(string=w2557) -> (number=w2556:dbl)  [unwired: 3 in, 1 out]
              n2089 = Fract/Exp String To Number(string=w2565) -> (number=w2564:dbl)  [unwired: 3 in, 1 out]
              n2090 = Fract/Exp String To Number(string=w2580) -> (number=w2576:dbl)  [unwired: 3 in, 1 out]
              n2091 = Fract/Exp String To Number(string=w2583) -> (number=w2574:dbl)  [unwired: 3 in, 1 out]
              n2092 = Fract/Exp String To Number(string=w2569) -> (number=w2572:dbl)  [unwired: 3 in, 1 out]
              n2093 = Add(x=w2572, y=0.0) -> (x+y=w2568:dbl)
            }
            n2094 = for {
              N: w2460 -> [_]
              tunnel: w2467 -> [w2515]
              tunnel: w2466 -> [w2514]
              tunnel: [w2504] -> w2420 mode=indexing
              tunnel: [w2503] -> w2413 mode=indexing
              tunnel: w2457 -> [_]
              tunnel: [w2492] -> w2418 mode=indexing
              tunnel: [w2497] -> w2415 mode=indexing
              tunnel: [w2493] -> w2405 mode=indexing
              tunnel: [w2488] -> w2380 mode=indexing
              tunnel: [w2484] -> w2361 mode=indexing
              tunnel: [w2479] -> w2321 mode=indexing
              (unwired) 1.0 ("x")
              (unwired) TRUE ("line mode (F)")
              n2095 = Read from Text File "Read File"(file (use dialog)=w2515, error in=w2514) -> (text=w2480:string)  [unwired: 2 in, 3 out]
              n2096 = local write "String 12"(w2480) -> ()
              n2097 = String Subset(string=w2480, offset (0)=85, length (rest)=9 ("length (rest)")) -> (substring=w2482:string)
              n2098 = String Subset(string=w2480, offset (0)=35, length (rest)=9 ("length (rest)")) -> (substring=w2505:string)
              n2099 = String Subset(string=w2480, offset (0)=55, length (rest)=9 ("length (rest)")) -> (substring=w2490:string)
              n2100 = String Subset(string=w2480, offset (0)=25, length (rest)=9 ("length (rest)")) -> (substring=w2486:string)
              n2101 = String Subset(string=w2480, offset (0)=45, length (rest)=9 ("length (rest)")) -> (substring=w2495:string)
              n2102 = String Subset(string=w2480, offset (0)=15, length (rest)=9 ("length (rest)")) -> (substring=w2511:string)
              n2103 = String Subset(string=w2480, offset (0)=0, length (rest)=14 ("length (rest)")) -> (substring=w2508:string)
              n2104 = String Subset(string=w2480, offset (0)=65, length (rest)=9 ("length (rest)")) -> (substring=w2498:string)
              n2105 = Fract/Exp String To Number(string=w2482) -> (number=w2479:dbl)  [unwired: 3 in, 1 out]
              n2106 = Fract/Exp String To Number(string=w2505) -> (number=w2503:dbl)  [unwired: 3 in, 1 out]
              n2107 = Fract/Exp String To Number(string=w2490) -> (number=w2488:dbl)  [unwired: 3 in, 1 out]
              n2108 = Fract/Exp String To Number(string=w2486) -> (number=w2484:dbl)  [unwired: 3 in, 1 out]
              n2109 = Fract/Exp String To Number(string=w2495) -> (number=w2493:dbl)  [unwired: 3 in, 1 out]
              n2110 = Fract/Exp String To Number(string=w2511) -> (number=w2492:dbl)  [unwired: 3 in, 1 out]
              n2111 = Fract/Exp String To Number(string=w2508) -> (number=w2504:dbl)  [unwired: 3 in, 1 out]
              n2112 = Fract/Exp String To Number(string=w2498) -> (number=w2501:dbl)  [unwired: 3 in, 1 out]
              n2113 = Add(x=w2501, y=0.0) -> (x+y=w2497:dbl)
            }
            n2114 = Delete From Array(array=w2363, index=0) -> (array with subset deleted=w2336:dbl[])  [unwired: 1 in, 1 out]
            n2115 = Delete From Array(array=w2426, index=0) -> (array with subset deleted=w2399:dbl[])  [unwired: 1 in, 1 out]
            n2116 = Delete From Array(array=w2406, index=0) -> (array with subset deleted=w2394:dbl[])  [unwired: 1 in, 1 out]
            n2117 = Delete From Array(array=w2424, index=0) -> (array with subset deleted=w2425:dbl[])  [unwired: 1 in, 1 out]
            n2118 = call-poly <vilib>:"Mean.vi"("X"=w2336) -> ("mean"=→"КОФ2 4":dbl)  [unwired: 1 out]
            n2119 = call-poly <vilib>:"Mean.vi"("X"=w2399) -> ("mean"=→"КОФ3":dbl)  [unwired: 1 out]
            n2120 = call-poly <vilib>:"Mean.vi"("X"=w2394) -> ("mean"=→"CP3":dbl)  [unwired: 1 out]
            n2121 = Delete From Array(array=w2388, index=0) -> (array with subset deleted=w2315:dbl[])  [unwired: 1 in, 1 out]
            n2122 = Delete From Array(array=w2327, index=0) -> (array with subset deleted=w2314:dbl[])  [unwired: 1 in, 1 out]
            n2123 = Delete From Array(array=w2367, index=0) -> (array with subset deleted=w2338:dbl[])  [unwired: 1 in, 1 out]
            n2124 = Delete From Array(array=w2445, index=0) -> (array with subset deleted=w2400:dbl[])  [unwired: 1 in, 1 out]
            n2125 = Delete From Array(array=w2411, index=0) -> (array with subset deleted=w2396:dbl[])  [unwired: 1 in, 1 out]
            "array w/ subset deleted" <- w2396
            n2126 = Delete From Array(array=w2442, index=0) -> (array with subset deleted=w2443:dbl[])  [unwired: 1 in, 1 out]
            n2127 = call-poly <vilib>:"Mean.vi"("X"=w2338) -> ("mean"=→"КОФ2 2":dbl)  [unwired: 1 out]
            n2128 = call-poly <vilib>:"Mean.vi"("X"=w2400) -> ("mean"=→"КОФ1":dbl)  [unwired: 1 out]
            n2129 = Bundle "Bundle"(w2315, w2314) -> (w2320:cluster{dbl[], dbl[]})  [unwired: 1 in]
            n2130 = Bundle "Bundle"(w2315, w2443) -> (w2307:cluster{dbl[], dbl[]})  [unwired: 1 in]
            n2131 = Delete From Array(array=w2322, index=0) -> (array with subset deleted=w2310:dbl[])  [unwired: 1 in, 1 out]
            n2132 = Delete From Array(array=w2323, index=0) -> (array with subset deleted=w2312:dbl[])  [unwired: 1 in, 1 out]
            n2133 = Delete From Array(array=w2433, index=0) -> (array with subset deleted=w2434:dbl[])  [unwired: 1 in, 1 out]
            n2134 = Delete From Array(array=w2321, index=0) -> (array with subset deleted=w2308:dbl[])  [unwired: 1 in, 1 out]
            n2135 = Delete From Array(array=w2415, index=0) -> (array with subset deleted=w2416:dbl[])  [unwired: 1 in, 1 out]
            n2136 = Delete From Array(array=w2440, index=0) -> (array with subset deleted=w2346:dbl[])  [unwired: 1 in, 1 out]
            n2137 = Delete From Array(array=w2386, index=0) -> (array with subset deleted=w2342:dbl[])  [unwired: 1 in, 1 out]
            n2138 = Delete From Array(array=w2422, index=0) -> (array with subset deleted=w2344:dbl[])  [unwired: 1 in, 1 out]
            n2139 = Delete From Array(array=w2382, index=0) -> (array with subset deleted=w2340:dbl[])  [unwired: 1 in, 1 out]
            n2140 = Delete From Array(array=w2431, index=0) -> (array with subset deleted=w2345:dbl[])  [unwired: 1 in, 1 out]
            n2141 = Delete From Array(array=w2384, index=0) -> (array with subset deleted=w2341:dbl[])  [unwired: 1 in, 1 out]
            n2142 = Delete From Array(array=w2365, index=0) -> (array with subset deleted=w2337:dbl[])  [unwired: 1 in, 1 out]
            n2143 = Delete From Array(array=w2409, index=0) -> (array with subset deleted=w2395:dbl[])  [unwired: 1 in, 1 out]
            n2144 = Delete From Array(array=w2436, index=0) -> (array with subset deleted=w2397:dbl[])  [unwired: 1 in, 1 out]
            n2145 = Delete From Array(array=w2413, index=0) -> (array with subset deleted=w2343:dbl[])  [unwired: 1 in, 1 out]
            n2146 = Delete From Array(array=w2380, index=0) -> (array with subset deleted=w2339:dbl[])  [unwired: 1 in, 1 out]
            n2147 = Delete From Array(array=w2361, index=0) -> (array with subset deleted=w2335:dbl[])  [unwired: 1 in, 1 out]
            n2148 = Delete From Array(array=w2405, index=0) -> (array with subset deleted=w2393:dbl[])  [unwired: 1 in, 1 out]
            n2149 = Delete From Array(array=w2418, index=0) -> (array with subset deleted=w2398:dbl[])  [unwired: 1 in, 1 out]
            n2150 = Delete From Array(array=w2428, index=0) -> (array with subset deleted=w2311:dbl[])  [unwired: 1 in, 1 out]
            n2151 = Delete From Array(array=w2438, index=0) -> (array with subset deleted=w2313:dbl[])  [unwired: 1 in, 1 out]
            n2152 = Delete From Array(array=w2420, index=0) -> (array with subset deleted=w2309:dbl[])  [unwired: 1 in, 1 out]
            n2153 = Bundle "Bundle"(w2315, w2346) -> (w2333:cluster{dbl[], dbl[]})  [unwired: 1 in]
            n2154 = Bundle "Bundle"(w2315, w2400) -> (w2334:cluster{dbl[], dbl[]})  [unwired: 1 in]